vi "HFRR ADV v044.vi"() -> ()   [LabVIEW 2025] (continued)
              n2263 = Fract/Exp String To Number(string=w2652) -> (number=w2648:dbl)  [unwired: 3 in, 1 out]
              n2264 = Fract/Exp String To Number(string=w2642) -> (number=w2645:dbl)  [unwired: 3 in, 1 out]
              n2265 = Add(x=w2645, y=0.0) -> (x+y=w2641:dbl)
            }
            n2266 = Delete From Array(array=w2507, index=0) -> (array with subset deleted=w2480:dbl[])  [unwired: 1 in, 1 out]
            n2267 = Delete From Array(array=w2570, index=0) -> (array with subset deleted=w2543:dbl[])  [unwired: 1 in, 1 out]
            n2268 = Delete From Array(array=w2550, index=0) -> (array with subset deleted=w2538:dbl[])  [unwired: 1 in, 1 out]
            n2269 = Delete From Array(array=w2568, index=0) -> (array with subset deleted=w2569:dbl[])  [unwired: 1 in, 1 out]
            n2270 = call-poly <vilib>:"Mean.vi"("X"=w2480) -> ("mean"=→"КОФ2 4":dbl)  [unwired: 1 out]
            n2271 = call-poly <vilib>:"Mean.vi"("X"=w2543) -> ("mean"=→"КОФ3":dbl)  [unwired: 1 out]
            n2272 = call-poly <vilib>:"Mean.vi"("X"=w2538) -> ("mean"=→"CP3":dbl)  [unwired: 1 out]
            n2273 = Delete From Array(array=w2532, index=0) -> (array with subset deleted=w2459:dbl[])  [unwired: 1 in, 1 out]
            n2274 = Delete From Array(array=w2471, index=0) -> (array with subset deleted=w2458:dbl[])  [unwired: 1 in, 1 out]
            n2275 = Delete From Array(array=w2511, index=0) -> (array with subset deleted=w2482:dbl[])  [unwired: 1 in, 1 out]
            n2276 = Delete From Array(array=w2589, index=0) -> (array with subset deleted=w2544:dbl[])  [unwired: 1 in, 1 out]
            n2277 = Delete From Array(array=w2555, index=0) -> (array with subset deleted=w2540:dbl[])  [unwired: 1 in, 1 out]
            "array w/ subset deleted" <- w2540
            n2278 = Delete From Array(array=w2586, index=0) -> (array with subset deleted=w2587:dbl[])  [unwired: 1 in, 1 out]
            n2279 = call-poly <vilib>:"Mean.vi"("X"=w2482) -> ("mean"=→"КОФ2 2":dbl)  [unwired: 1 out]
            n2280 = call-poly <vilib>:"Mean.vi"("X"=w2544) -> ("mean"=→"КОФ1":dbl)  [unwired: 1 out]
            n2281 = Bundle "Bundle"(w2459, w2458) -> (w2464:cluster{dbl[], dbl[]})  [unwired: 1 in]
            n2282 = Bundle "Bundle"(w2459, w2587) -> (w2451:cluster{dbl[], dbl[]})  [unwired: 1 in]
            n2283 = Delete From Array(array=w2466, index=0) -> (array with subset deleted=w2454:dbl[])  [unwired: 1 in, 1 out]
            n2284 = Delete From Array(array=w2467, index=0) -> (array with subset deleted=w2456:dbl[])  [unwired: 1 in, 1 out]
            n2285 = Delete From Array(array=w2577, index=0) -> (array with subset deleted=w2578:dbl[])  [unwired: 1 in, 1 out]
            n2286 = Delete From Array(array=w2465, index=0) -> (array with subset deleted=w2452:dbl[])  [unwired: 1 in, 1 out]
            n2287 = Delete From Array(array=w2559, index=0) -> (array with subset deleted=w2560:dbl[])  [unwired: 1 in, 1 out]
            n2288 = Delete From Array(array=w2584, index=0) -> (array with subset deleted=w2490:dbl[])  [unwired: 1 in, 1 out]
            n2289 = Delete From Array(array=w2530, index=0) -> (array with subset deleted=w2486:dbl[])  [unwired: 1 in, 1 out]
            n2290 = Delete From Array(array=w2566, index=0) -> (array with subset deleted=w2488:dbl[])  [unwired: 1 in, 1 out]
            n2291 = Delete From Array(array=w2526, index=0) -> (array with subset deleted=w2484:dbl[])  [unwired: 1 in, 1 out]
            n2292 = Delete From Array(array=w2575, index=0) -> (array with subset deleted=w2489:dbl[])  [unwired: 1 in, 1 out]
            n2293 = Delete From Array(array=w2528, index=0) -> (array with subset deleted=w2485:dbl[])  [unwired: 1 in, 1 out]
            n2294 = Delete From Array(array=w2509, index=0) -> (array with subset deleted=w2481:dbl[])  [unwired: 1 in, 1 out]
            n2295 = Delete From Array(array=w2553, index=0) -> (array with subset deleted=w2539:dbl[])  [unwired: 1 in, 1 out]
            n2296 = Delete From Array(array=w2580, index=0) -> (array with subset deleted=w2541:dbl[])  [unwired: 1 in, 1 out]
            n2297 = Delete From Array(array=w2557, index=0) -> (array with subset deleted=w2487:dbl[])  [unwired: 1 in, 1 out]
            n2298 = Delete From Array(array=w2524, index=0) -> (array with subset deleted=w2483:dbl[])  [unwired: 1 in, 1 out]
            n2299 = Delete From Array(array=w2505, index=0) -> (array with subset deleted=w2479:dbl[])  [unwired: 1 in, 1 out]
            n2300 = Delete From Array(array=w2549, index=0) -> (array with subset deleted=w2537:dbl[])  [unwired: 1 in, 1 out]
            n2301 = Delete From Array(array=w2562, index=0) -> (array with subset deleted=w2542:dbl[])  [unwired: 1 in, 1 out]
            n2302 = Delete From Array(array=w2572, index=0) -> (array with subset deleted=w2455:dbl[])  [unwired: 1 in, 1 out]
            n2303 = Delete From Array(array=w2582, index=0) -> (array with subset deleted=w2457:dbl[])  [unwired: 1 in, 1 out]
            n2304 = Delete From Array(array=w2564, index=0) -> (array with subset deleted=w2453:dbl[])  [unwired: 1 in, 1 out]
            n2305 = Bundle "Bundle"(w2459, w2490) -> (w2477:cluster{dbl[], dbl[]})  [unwired: 1 in]
            n2306 = Bundle "Bundle"(w2459, w2544) -> (w2478:cluster{dbl[], dbl[]})  [unwired: 1 in]
            n2307 = Bundle "Bundle"(w2490, w2486) -> (w2492:cluster{dbl[], dbl[]})  [unwired: 1 in]
            n2308 = Bundle "Bundle"(w2455, w2454) -> (w2462:cluster{dbl[], dbl[]})  [unwired: 1 in]
            n2309 = Bundle "Bundle"(w2488, w2484) -> (w2494:cluster{dbl[], dbl[]})  [unwired: 1 in]
            n2310 = Bundle "Bundle"(w2455, w2488) -> (w2598:cluster{dbl[], dbl[]})  [unwired: 1 in]
            n2311 = Bundle "Bundle"(w2455, w2484) -> (w2522:cluster{dbl[], dbl[]})  [unwired: 1 in]
            n2312 = Bundle "Bundle"(w2455, w2543) -> (w2608:cluster{dbl[], dbl[]})  [unwired: 1 in]
            n2313 = Bundle "Bundle"(w2455, w2538) -> (w2546:cluster{dbl[], dbl[]})  [unwired: 1 in]
            n2314 = Bundle "Bundle"(w2455, w2569) -> (w2593:cluster{dbl[], dbl[]})  [unwired: 1 in]
            n2315 = Bundle "Bundle"(w2489, w2485) -> (w2493:cluster{dbl[], dbl[]})  [unwired: 1 in]
            n2316 = Bundle "Bundle"(w2457, w2456) -> (w2463:cluster{dbl[], dbl[]})  [unwired: 1 in]
            n2317 = Bundle "Bundle"(w2457, w2489) -> (w2600:cluster{dbl[], dbl[]})  [unwired: 1 in]
            n2318 = Bundle "Bundle"(w2457, w2485) -> (w2523:cluster{dbl[], dbl[]})  [unwired: 1 in]
            n2319 = Bundle "Bundle"(w2457, w2539) -> (w2547:cluster{dbl[], dbl[]})  [unwired: 1 in]
            n2320 = Bundle "Bundle"(w2457, w2541) -> (w2609:cluster{dbl[], dbl[]})  [unwired: 1 in]
            n2321 = Bundle "Bundle"(w2457, w2578) -> (w2591:cluster{dbl[], dbl[]})  [unwired: 1 in]
            n2322 = Bundle "Bundle"(w2487, w2483) -> (w2495:cluster{dbl[], dbl[]})  [unwired: 1 in]
            n2323 = Bundle "Bundle"(w2453, w2452) -> (w2461:cluster{dbl[], dbl[]})  [unwired: 1 in]
            n2324 = Bundle "Bundle"(w2453, w2487) -> (w2599:cluster{dbl[], dbl[]})  [unwired: 1 in]
            n2325 = Bundle "Bundle"(w2453, w2483) -> (w2521:cluster{dbl[], dbl[]})  [unwired: 1 in]
            n2326 = Bundle "Bundle"(w2453, w2537) -> (w2545:cluster{dbl[], dbl[]})  [unwired: 1 in]
            n2327 = Bundle "Bundle"(w2453, w2542) -> (w2607:cluster{dbl[], dbl[]})  [unwired: 1 in]
            n2328 = Bundle "Bundle"(w2453, w2560) -> (w2592:cluster{dbl[], dbl[]})  [unwired: 1 in]
            n2329 = call-poly <vilib>:"Mean.vi"("X"=w2540) -> ("mean"=→"CP1":dbl)  [unwired: 1 out]
            n2330 = call-poly <vilib>:"Mean.vi"("X"=w2481) -> ("mean"=→"КОФ2 3":dbl)  [unwired: 1 out]
            n2331 = call-poly <vilib>:"Mean.vi"("X"=w2539) -> ("mean"=→"CP2":dbl)  [unwired: 1 out]
            n2332 = call-poly <vilib>:"Mean.vi"("X"=w2541) -> ("mean"=→"КОФ2":dbl)  [unwired: 1 out]
            n2333 = call-poly <vilib>:"Mean.vi"("X"=w2479) -> ("mean"=→"КОФ2 5":dbl)  [unwired: 1 out]
            n2334 = call-poly <vilib>:"Mean.vi"("X"=w2537) -> ("mean"=→"CP4":dbl)  [unwired: 1 out]
            n2335 = call-poly <vilib>:"Mean.vi"("X"=w2542) -> ("mean"=→"КОФ4":dbl)  [unwired: 1 out]
            n2336 = Bundle "Bundle"(w2459, w2486) -> (w2450:cluster{dbl[], dbl[]})  [unwired: 1 in]
            n2337 = Bundle "Bundle"(w2459, w2540) -> (w2473:cluster{dbl[], dbl[]})  [unwired: 1 in]
            n2338 = Build Array "Build Array"(w2450, w2473) -> (w2476:cluster{dbl[], dbl[]}[])
            "XY Graph 17" <- w2476
            n2339 = Build Array "Build Array"(w2464, w2463, w2462, w2461) -> (→"Frequency ( Hz )":cluster{dbl[], dbl[]}[])
            n2340 = Build Array "Build Array"(w2492, w2493, w2494, w2495) -> (→"Air Temp ( °C ) vs Humidity ( % RH )":cluster{dbl[], dbl[]}[])
            n2341 = Build Array "Build Array"(w2477, w2600, w2598, w2599) -> (→"Air Temperature  ( °C )":cluster{dbl[], dbl[]}[])
            n2342 = Build Array "Build Array"(w2450, w2523, w2522, w2521) -> (→"Humidity ( %RH )":cluster{dbl[], dbl[]}[])
            n2343 = Build Array "Build Array"(w2478, w2609, w2608, w2607) -> (→"Coefficient Of Friction":cluster{dbl[], dbl[]}[])
            n2344 = Build Array "Build Array"(w2473, w2547, w2546, w2545) -> (→"Sample Temperature ( °C )":cluster{dbl[], dbl[]}[])
            n2345 = Build Array "Build Array"(w2451, w2591, w2593, w2592) -> (→"XY Graph 13":cluster{dbl[], dbl[]}[])
            n2346 = Bundle "Bundle"(w2459, w2482) -> (w2504:cluster{dbl[], dbl[]})  [unwired: 1 in]
            n2347 = Bundle "Bundle"(w2455, w2480) -> (w2502:cluster{dbl[], dbl[]})  [unwired: 1 in]
            n2348 = Bundle "Bundle"(w2457, w2481) -> (w2503:cluster{dbl[], dbl[]})  [unwired: 1 in]
            n2349 = Bundle "Bundle"(w2453, w2479) -> (w2501:cluster{dbl[], dbl[]})  [unwired: 1 in]
            n2350 = Build Array "Build Array"(w2504, w2503, w2502, w2501) -> (→"Stroke ( mm )":cluster{dbl[], dbl[]}[])
            n2351 = local write "XY Graph 16"(w2476) -> ()
          }
          frame #2 {
          }
          frame #3 {
            n2352 = local write "Numeric 8"(0 ("Numeric 8")) -> ()
            n2353 = local write "Numeric 11"(0 ("Numeric 11")) -> ()
            n2354 = local write "Numeric 12"(0 ("Numeric 12")) -> ()
            n2355 = local write "Numeric 13"(0 ("Numeric 13")) -> ()
            n2356 = property on="OPEN" class="Bool (strict)"("Visible"=TRUE) -> ()  [unwired: 2 in, 2 out]
            n2357 = local read "String Control 2"() -> (w2776:string)
            n2358 = local read "String Control 4"() -> (w2775:string)
            n2359 = local read "String Control 6"() -> (w2774:string)
            n2360 = local read "String Control 8"() -> (w2773:string)
            n2361 = Match Pattern(string=w2776, regular expression="Samples / cycle :- ") -> (after substring=w2790:string)  [unwired: 1 in, 3 out]
            n2362 = Match Pattern(string=w2776, regular expression="Frequency :- ") -> (after substring=w2809:string)  [unwired: 1 in, 3 out]
            n2363 = Match Pattern(string=w2775, regular expression="Samples / cycle :- ") -> (after substring=w2786:string)  [unwired: 1 in, 3 out]
            n2364 = Match Pattern(string=w2775, regular expression="Frequency :- ") -> (after substring=w2804:string)  [unwired: 1 in, 3 out]
            n2365 = Match Pattern(string=w2774, regular expression="Samples / cycle :- ") -> (after substring=w2782:string)  [unwired: 1 in, 3 out]
            n2366 = Match Pattern(string=w2774, regular expression="Frequency :- ") -> (after substring=w2799:string)  [unwired: 1 in, 3 out]
            n2367 = Match Pattern(string=w2773, regular expression="Samples / cycle :- ") -> (after substring=w2778:string)  [unwired: 1 in, 3 out]
            n2368 = Match Pattern(string=w2773, regular expression="Frequency :- ") -> (after substring=w2794:string)  [unwired: 1 in, 3 out]
            n2369 = String Subset(string=w2790, length (rest)=6 ("length (rest)")) -> (substring=w2792:string)  [unwired: 1 in]
            n2370 = String Subset(string=w2809, length (rest)=9 ("length (rest)")) -> (substring=w2811:string)  [unwired: 1 in]
            n2371 = String Subset(string=w2786, length (rest)=6 ("length (rest)")) -> (substring=w2788:string)  [unwired: 1 in]
            n2372 = String Subset(string=w2804, length (rest)=9 ("length (rest)")) -> (substring=w2806:string)  [unwired: 1 in]
            n2373 = String Subset(string=w2782, length (rest)=6 ("length (rest)")) -> (substring=w2784:string)  [unwired: 1 in]
            n2374 = String Subset(string=w2799, length (rest)=9 ("length (rest)")) -> (substring=w2801:string)  [unwired: 1 in]
            n2375 = String Subset(string=w2778, length (rest)=6 ("length (rest)")) -> (substring=w2780:string)  [unwired: 1 in]
            n2376 = String Subset(string=w2794, length (rest)=9 ("length (rest)")) -> (substring=w2796:string)  [unwired: 1 in]
            n2377 = Fract/Exp String To Number(string=w2792) -> (number=w2772:dbl)  [unwired: 3 in, 1 out]
            n2378 = Fract/Exp String To Number(string=w2811) -> (number=w2812:dbl)  [unwired: 3 in, 1 out]
            n2379 = Fract/Exp String To Number(string=w2788) -> (number=w2771:dbl)  [unwired: 3 in, 1 out]
            n2380 = Fract/Exp String To Number(string=w2806) -> (number=w2807:dbl)  [unwired: 3 in, 1 out]
            n2381 = Fract/Exp String To Number(string=w2784) -> (number=w2770:dbl)  [unwired: 3 in, 1 out]
            n2382 = Fract/Exp String To Number(string=w2801) -> (number=w2802:dbl)  [unwired: 3 in, 1 out]
            n2383 = Fract/Exp String To Number(string=w2780) -> (number=w2769:dbl)  [unwired: 3 in, 1 out]
            n2384 = Fract/Exp String To Number(string=w2796) -> (number=w2797:dbl)  [unwired: 3 in, 1 out]
            n2385 = local write "sample1"(w2772) -> ()
            n2386 = local write "freq1"(w2812) -> ()
            n2387 = local write "sample2"(w2771) -> ()
            n2388 = local write "freq2"(w2807) -> ()
            n2389 = local write "sample3"(w2770) -> ()
            n2390 = local write "freq3"(w2802) -> ()
            n2391 = local write "sample4"(w2769) -> ()
            n2392 = local write "freq 4"(w2797) -> ()
          }
        }
      }
    }
    n2393 = case shown="True" w2370 {
      selector: w2370 -> [_ w2389]
      frame False {
      }
      frame True {
        n2394 = Not(x=w2389) -> (.not. x?=w2385:bool)
        n2395 = local write "service 3"(w2385) -> ()
        n2396 = local write "OPEN 6"(w2385) -> ()
        n2397 = call <vilib>:"System Exec.vi"("wait until completion? (T)"=TRUE, "command line"="C:\\LAB-IQ\\Scar View.exe") -> ("error out"=→"error out 5":errorcluster)  [unwired: 6 in, 3 out]
      }
    }
    n2398 = case shown="\"Acquire\", Default" w2379 {
      frame "Acquire", Default {
        # "Elapsed time\ncof\nstroke\nAir temp\nTemp\nHumidity"
        n2399 = disable-structure shown="Disabled" {
          frame Disabled {
            n2400 = local read "Flag"() -> (w3088:dbl)
            n2401 = local read "RUN"() -> (w3085:bool)
            n2402 = Not(x=w3085) -> (.not. x?=w3084:bool)
            n2403 = Equal?(x=w3088, y=10.0) -> (x = y?=w3086:bool)
            n2404 = And(x=w3086, y=w3084) -> (x .and. y?=w3083:bool)
            n2405 = case shown="True" w3083 {
              frame False {
              }
              frame True {
                w3089 = FALSE ("Heater Button")
                n2406 = local write "Humidity"(w3089) -> ()
                n2407 = local write "Heater Button"(w3089) -> ()
              }
            }
          }
          frame Enabled {
          }
        }
        n2408 = disable-structure shown="Disabled" {
          frame Disabled {
            n2409 = case shown="True" {
              selector: _ -> [_ _]
              frame False {
              }
              frame True {
                w3134 = TRUE ("Heater")
                n2410 = local write "Humidity"(w3134) -> ()
                n2411 = local write "Heater Button"(w3134) -> ()
                n2412 = local read "TEST STANDARD"() -> (w3137:T5)
                n2413 = local read "TEST STANDARD"() -> (w3132:T5)
                n2414 = Equal?(x=w3137, y=enum16{"ASTM D6079", "ISO 12156", "Custom"}."ISO 12156" ("Test Standard")) -> (x = y?=w3135:bool)
                n2415 = Equal?(x=w3132, y=enum16{"ASTM D6079", "ISO 12156", "Custom"}."ASTM D6079" ("Test Standard")) -> (x = y?=w3131:bool)
                n2416 = case shown="True" w3135 {
                  frame False {
                  }
                  frame True {
                    n2417 = local write "airtempflg"(FALSE ("airtempflg")) -> ()
                    n2418 = local write item#-1(TRUE ("Heater")) -> ()
                  }
                }
                n2419 = case shown="True" w3131 {
                  frame False {
                  }
                  frame True {
                    n2420 = local write "airtempflg"(TRUE ("airtempflg")) -> ()
                    n2421 = local write item#-1(FALSE ("Heater")) -> ()
                  }
                }
              }
            }
          }
          frame Enabled {
          }
        }
        n2422 = stacked-sequence {
          frame #0 {
            n2423 = case shown="True" "RST FF" {
              frame False {
              }
              frame True {
                w3151 = 0.0 ("X Scale.Range:Maximum")
                n2424 = property on="Frictional Force ( N )" class="WFChart (strict)"("XScale.Maximum"=600.0 ("X Scale.Range:Maximum"), "XScale.Minimum"=w3151, "YScale.Maximum"=10.0 ("Y Scale.Range:Maximum"), "YScale.Minimum"=w3151) -> ()  [unwired: 2 in, 2 out]
              }
            }
          }
          frame #1 {
            n2425 = case shown="True" "RST TEMP" {
              frame False {
              }
              frame True {
                n2426 = property on="Temperature ( Deg C )" class="WFChart (strict)"("XScale.Minimum"=0.0 ("X Scale.Range:Minimum"), "XScale.Maximum"=600.0 ("X Scale.Range:Maximum"), "YScale.Minimum"=0.0 ("Y Scale.Range:Minimum"), "YScale.Maximum"=100.0 ("Y Scale.Range:Maximum")) -> ()  [unwired: 2 in, 2 out]
              }
            }
          }
          frame #2 {
            n2427 = case shown="True" "RSTCOF" {
              frame False {
              }
              frame True {
                n2428 = property on="Coefficient of Friction" class="WFChart (strict)"("XScale.Minimum"=0.0 ("X Scale.Range:Minimum"), "XScale.Maximum"=600.0 ("X Scale.Range:Maximum"), "YScale.Maximum"=1.0 ("X Scale.Range:Minimum"), "YScale.Minimum"=0.0 ("X Scale.Range:Minimum")) -> ()  [unwired: 2 in, 2 out]
              }
            }
          }
          frame #3 {
            n2429 = case shown="True" "RSTCOF 2" {
              frame False {
              }
              frame True {
                (unwired) 100.0 ("Y Scale.Range:Maximum")
                (unwired) 0.0 ("Y Scale.Range:Minimum")
                (unwired) 600.0 ("X Scale.Range:Maximum")
                (unwired) 0.0 ("X Scale.Range:Minimum")
              }
            }
          }
          frame #4 {
            n2430 = case shown="True" "RSTCOF 3" {
              frame False {
              }
              frame True {
                n2431 = property on="Electrical Contact Resistance ( % )" class="WFChart (strict)"("XScale.Minimum"=0.0 ("X Scale.Range:Minimum"), "XScale.Maximum"=600.0 ("X Scale.Range:Maximum"), "YScale.Minimum"=0.0 ("Y Scale.Range:Minimum"), "YScale.Maximum"=100.0 ("Y Scale.Range:Maximum")) -> ()  [unwired: 2 in, 2 out]
              }
            }
          }
        }
        n2432 = local read "RUN"() -> (w3078:bool)
        n2433 = case shown="False" w3078 {
          frame False {
          }
          frame True {
          }
        }
        n2434 = local read "RUN"() -> (w3082:bool)
        n2435 = case shown="False" w3082 {
          tunnel: [FALSE ("TEST RUNNING") TRUE ("TEST RUNNING")] -> w3081
          frame False {
            w3170 = 0.0 ("Flag")
            n2436 = local write "Elapsed time"(0.0 ("elapsedtime")) -> ()
            n2437 = local write "Time Remaining"(w3170) -> ()
            n2438 = local write "Flag"(w3170) -> ()
            n2439 = local write "Remaining Time"(w3170) -> ()
          }
          frame True {
            n2440 = local write "Flag"(10.0 ("Flag")) -> ()
          }
        }
        n2441 = local read "AIR TEMP"() -> (w3076:dbl)
        n2442 = Greater Or Equal?(x=w3076, y=15.0) -> (x >= y?=w3077:bool)
        "powstat" <- w3077
        n2443 = case shown="True" "Save & Continue" {
          frame False {
          }
          frame True {
            n2444 = local read "USER ID"() -> (w3474:string)
            n2445 = local read "FILE"() -> (w3482:string)
            n2446 = String Length(string=w3482) -> (length=w3480:i32)
            n2447 = String Length(string=w3474) -> (length=w3477:i32)
            n2448 = Greater?(x=w3480, y=0) -> (0:w3479:bool)
            n2449 = Greater?(x=w3477, y=0) -> (0:w3476:bool)
            n2450 = And(x=w3479, y=w3476) -> (x .and. y?=w3475:bool)
            n2451 = case shown="True" w3475 {
              frame False {
                n2452 = stacked-sequence {
                  frame #0 {
                    n2453 = One Button Dialog(message="Please Enter a File Name and Operator ID to save data !", button name ("OK")="Ok") -> ()  [unwired: 1 out]
                  }
                  frame #1 {
                    n2454 = local write "Save & Continue"(FALSE ("OK Button")) -> ()
                  }
                }
                n2455 = local write "Save & Continue"(FALSE ("OK Button")) -> ()
              }
              frame True {
                n2456 = stacked-sequence {
                  frame #0 {
                    n2457 = local read "FILE"() -> (w3488:string)
                    n2458 = call "file check.vi"("file name in"=w3488) -> ("file name out"=w3487:string)  [unwired: 9 in, 1 out]
                    n2459 = call <vilib>:"Application Directory.vi"() -> ("Application Directory"=w3498:path)
                    n2460 = Build Path(base path=w3498, name or relative path="data") -> (appended path=w3497:path)
                    n2461 = call <vilib>:"Trim Whitespace.vi"("string"=w3487) -> ("trimmed string"=w3495:string)  [unwired: 1 in]
                    n2462 = call <vilib>:"Trim Whitespace.vi"("string"=w3487) -> ("trimmed string"=w3496:string)  [unwired: 1 in]
                    n2463 = List Folder(path=w3497) -> (folder names=w3493:string[])  [unwired: 3 in, 3 out]
                    n2464 = Match Pattern(string=w3495, regular expression="_(") -> (before substring=w3492:string)  [unwired: 1 in, 3 out]
                    n2465 = for {
                      tunnel: w3493 -> [w3507] mode=indexing
                      tunnel: w3492 -> [w3505]
                      shift-right: [w3503] -> w3490
                      shift-left: bool[] [] -> [w3504]
                      n2466 = Match Pattern(string=w3507, regular expression="_(") -> (before substring=w3506:string)  [unwired: 1 in, 3 out]
                      n2467 = Equal?(x=w3506, y=w3505) -> (x = y?=w3502:bool)
                      n2468 = case shown="True" w3502 {
                        tunnel: w3502 -> [_ w3510]
                        tunnel: w3504 -> [w3509 w3512]
                        tunnel: [w3509 w3511] -> w3503
                        frame False {
                        }
                        frame True {
                          n2469 = Insert Into Array(array=w3512, new element=w3510) -> (w3511:bool[])  [unwired: 1 in]
                        }
                      }
                    }
                    n2470 = Equal?(x=w3493, y=w3492) -> (x = y?=w3501:bool[])
                    n2471 = Or Array Elements(Boolean array=w3501) -> (logical OR=w3500:bool)
                    n2472 = Array Size(array=w3490) -> (size(s)=w3489:i32)
                    n2473 = case shown="True" w3500 {
                      tunnel: w3496 -> [_ w3520]
                      tunnel: w3489 -> [_ w3513]
                      frame False {
                      }
                      frame True {
                        n2474 = Number To Decimal String(number=w3513) -> (decimal integer string=w3516:string)  [unwired: 1 in]
                        n2475 = Search/Split String(string=w3520, search string/char (-)="_(" ("regular expression")) -> (substring before match=w3518:string)  [unwired: 1 in, 2 out]
                        n2476 = Concatenate Strings(w3518, "_(" ("regular expression"), w3516, ")" ("regular expression")) -> (w3514:string)
                        n2477 = local write "FILE"(w3514) -> ()
                      }
                    }
                  }
                  frame #1 {
                    w3523 = 0.0
                    w3536 = cluster{"y":dbl, dbl, "y":dbl}[] [] ("History Data")
                    w3537 = FALSE ("Heater Button")
                    (unwired) ")!" ("string")
                    (unwired) ")" ("string")
                    w3535 = dbl[] [] ("History Data")
                    w3541 = "\r"
                    # "C:\\WinDucom\\Data\\"
                    # "C:\\LAB-IQ-NXT\\data"
                    n2478 = local write "Humidity ( %RH )"(w3523) -> ()
                    n2479 = local write "Frequency ( Hz )"(w3523) -> ()
                    n2480 = local write "Stroke 3"(w3523) -> ()
                    n2481 = local write "speedop"(0.0 ("PIDclk 2")) -> ()
                    n2482 = local write "Set Temp 2"(65.0 ("Set Temp 2")) -> ()
                    n2483 = local write "AIR TEMP"(w3523) -> ()
                    n2484 = local write "clk"(0.0 ("clk")) -> ()
                    n2485 = local write "Stroke 4"(w3523) -> ()
                    n2486 = local write "COF 2"(w3523) -> ()
                    n2487 = local write "TEMP"(w3523) -> ()
                    n2488 = local write "ecr 3"(w3523) -> ()
                    n2489 = local write "FF 3"(w3523) -> ()
                    n2490 = local write "FF 2"(w3523) -> ()
                    n2491 = property on="Coefficient of Friction" class="WFChart (strict)"("History Data"=w3535) -> ()  [unwired: 2 in, 2 out]
                    n2492 = property on="Coefficient of Friction" class="WFChart (strict)"("History Data"=w3535) -> ()  [unwired: 2 in, 2 out]
                    n2493 = property on="Frictional Force ( N )" class="WFChart (strict)"("History Data"=w3535) -> ()  [unwired: 2 in, 2 out]
                    n2494 = property on="Electrical Contact Resistance ( % )" class="WFChart (strict)"("History Data"=w3535) -> ()  [unwired: 2 in, 2 out]
                    n2495 = property on="Electrical Contact Resistance ( % )" class="WFChart (strict)"("History Data"=w3535) -> ()  [unwired: 2 in, 2 out]
                    n2496 = property on="Temperature ( Deg C )" class="WFChart (strict)"("History Data"=w3535) -> ()  [unwired: 2 in, 2 out]
                    n2497 = property on="Frictional Force ( N )" class="WFChart (strict)"("History Data"=w3535) -> ()  [unwired: 2 in, 2 out]
                    n2498 = property on="Coefficient of Friction" class="WFChart (strict)"("History Data"=w3535) -> ()  [unwired: 2 in, 2 out]
                    n2499 = property on="Frictional Force ( N )" class="WFChart (strict)"("History Data"=w3535) -> ()  [unwired: 2 in, 2 out]
                    n2500 = property on="Electrical Contact Resistance ( % )" class="WFChart (strict)"("History Data"=w3535) -> ()  [unwired: 2 in, 2 out]
                    n2501 = property on="Temperature ( Deg C )" class="WFChart (strict)"("History Data"=w3535) -> ()  [unwired: 2 in, 2 out]
                    n2502 = property on="Stroke ( mm )" class="WFChart (strict)"("History Data"=w3536) -> ()  [unwired: 2 in, 2 out]
                    n2503 = property on="Stroke ( mm )" class="WFChart (strict)"("History Data"=w3536) -> ()  [unwired: 2 in, 2 out]
                    n2504 = local write "Humidity"(w3537) -> ()
                    n2505 = local write "Heater Button"(w3537) -> ()
                    n2506 = local read "FILE"() -> (w3531:string)
                    n2507 = disable-structure shown="Enabled" {
                      disable-tunnel: [w3575 _] -> w3522
                      frame Enabled {
                        n2508 = local read "NORMAL LOAD"() -> (w3575:dbl)
                      }
                      frame Disabled {
                      }
                    }
                    n2509 = call "file check.vi"("file name in"=w3531) -> ("error out"=w3534:errorcluster, "file name out"=w3528:string)  [unwired: 9 in]
                    n2510 = call "FILE PATH CREATION.vi"("error in"=w3534, "FILE NAME :"=w3528) -> ("FILE OUT"=w3527:path)  [unwired: 8 in, 1 out]
                    n2511 = Concatenate Strings(w3528, ".dgf" ("Substring")) -> (w3533:string)
                    n2512 = Concatenate Strings(w3528, ".duf" ("Substring")) -> (w3529:string)
                    n2513 = Multiply(x=w3522, y=1.0) -> (x*y=w3554:dbl)
                    n2514 = Build Path(base path=w3527, name or relative path=w3533) -> (appended path=w3526:path)
                    n2515 = Build Path(base path=w3527, name or relative path=w3529) -> (appended path=w3525:path)
                    n2516 = Number To Fractional String(number=w3554, width (-)=i16 5, precision (6)=i16 2) -> (F-format string=w3562:string)  [unwired: 1 in]
                    n2517 = local read "tested by"() -> (w3521:string)
                    n2518 = local read "Fuel Discription :"() -> (w3550:string)
                    n2519 = local read "Batch Ref Num :"() -> (w3539:string)
                    n2520 = Get Date/Time String(date format (0)=enum16{"short", "long", "abbreviated"}."short") -> (date string=w3573:string, time string=w3570:string)  [unwired: 2 in]
                    n2521 = local read "Remarks :"() -> (w3549:string)
                    n2522 = Concatenate Strings("Load :- " ("Substring"), w3562, " grams ," ("Substring")) -> (w3561:string)
                    n2523 = local read "String 41"() -> (w3542:string)
                    n2524 = Concatenate Strings(w3550) -> (w3551:string)
                    n2525 = Concatenate Strings(w3539) -> (w3538:string)
                    n2526 = Concatenate Strings(w3521) -> (w3545:string)
                    n2527 = Concatenate Strings("(" ("Substring"), w3573, ")" ("Substring"), w3570) -> (w3544:string)
                    "concatenated string" <- w3544
                    n2528 = Concatenate Strings(w3549, "," ("string")) -> (w3548:string)
                    n2529 = Concatenate Strings("  TIME;      COF;       STROKE;     AIR TEMP;  TEMP;  HUMIDITY;  ECR; PID-OUT; FREQUENCY" ("Substring"), "\r") -> (w3557:string)
                    n2530 = Concatenate Strings(w3542, w3541, "Fuel Discription :-" ("Substring"), w3551, w3541, w3561, w3541, "Batch Ref Num :-" ("Substring"), w3538, w3541, " Remarks :- " ("Substring"), w3548, w3541, " Date :- " ("Substring"), w3544, w3541, "Tested By :-" ("Substring"), w3545) -> (w3555:string)
                    "REMARKS" <- w3555
                    n2531 = call <vilib>:"Write Characters To File.vi"("append to file? (new file:F)"=FALSE, "character string"=w3557, "file path (dialog if empty)"=w3526) -> ()  [unwired: 2 in, 1 out]
                    n2532 = call <vilib>:"Write Characters To File.vi"("append to file? (new file:F)"=FALSE, "character string"=w3555, "file path (dialog if empty)"=w3525) -> ()  [unwired: 2 in, 1 out]
                  }
                  frame #2 {
                    n2533 = local write "Cycles elapsed"(0 ("Cycles elapsed")) -> ()
                    n2534 = local write "cyclecount"(0 ("cyclecount")) -> ()
                    n2535 = local write "Save & Continue"(FALSE ("OK")) -> ()
                    n2536 = local write "autostrtflg"(TRUE ("autostrtflg")) -> ()
                    n2537 = local write "Save"(FALSE ("Save")) -> ()
                    n2538 = Get Date/Time In Seconds() -> (seconds since 1Jan1904=w3580:timestamp)
                    n2539 = To Double Precision Float(number=w3580) -> (double precision float=w3579:dbl)
                    n2540 = local write "acq timer"(w3579) -> ()
                    n2541 = One Button Dialog(message="Please ensure sample is mounted properly and machine is ready in all aspects for testing !", button name ("OK")="Ok") -> ()  [unwired: 1 out]
                  }
                  frame #3 {
                    n2542 = stacked-sequence {
                      frame #0 {
                        n2543 = local write "Main Dashboard Buttons"(T1."Dashboard" ("Main Dashboard Buttons")) -> ()
                        n2544 = local write "Main Tab"(T4."Acquire" ("Main Tab")) -> ()
                      }
                      frame #1 {
                        n2545 = local write "EVENT LOG"("" ("EVENT LOG")) -> ()
                      }
                      frame #2 {
                        n2546 = Wait (ms)(milliseconds to wait=u32 50) -> ()  [unwired: 1 out]
                      }
                      frame #3 {
                        n2547 = disable-structure shown="Disabled" {
                          frame Disabled {
                            n2548 = local read "EVENT LOG"() -> (w3592:string)
                            n2549 = call "Event Log.vi"("Content"="Test Details", "EVENT LOG"=w3592) -> ("EVENT LOG"=w3591:string)  [unwired: 8 in, 1 out]
                            n2550 = local write "EVENT LOG"(w3591) -> ()
                          }
                          frame Enabled {
                          }
                        }
                      }
                      frame #4 {
                        n2551 = Wait (ms)(milliseconds to wait=u32 50) -> ()  [unwired: 1 out]
                      }
                      frame #5 {
                        n2552 = local read "FILE"() -> (w3594:string)
                        n2553 = Concatenate Strings("File Name :" ("Content"), w3594) -> (w3595:string)
                        n2554 = local read "EVENT LOG"() -> (w3598:string)
                        n2555 = call "Event Log.vi"("Content"=w3595, "EVENT LOG"=w3598) -> ("EVENT LOG"=w3597:string)  [unwired: 8 in, 1 out]
                        n2556 = local write "EVENT LOG"(w3597) -> ()
                      }
                      frame #6 {
                        n2557 = Wait (ms)(milliseconds to wait=u32 50) -> ()  [unwired: 1 out]
                      }
                      frame #7 {
                        n2558 = local read "Batch Ref Num :"() -> (w3600:string)
                        n2559 = Concatenate Strings("Batch Ref No :" ("Content"), w3600) -> (w3601:string)
                        n2560 = local read "EVENT LOG"() -> (w3604:string)
                        n2561 = call "Event Log.vi"("Content"=w3601, "EVENT LOG"=w3604) -> ("EVENT LOG"=w3603:string)  [unwired: 8 in, 1 out]
                        n2562 = local write "EVENT LOG"(w3603) -> ()
                      }
                      frame #8 {
                        n2563 = Wait (ms)(milliseconds to wait=u32 50) -> ()  [unwired: 1 out]
                      }
                      frame #9 {
                        n2564 = local read "tested by"() -> (w3606:string)
                        n2565 = Concatenate Strings("Tested By :" ("Content"), w3606) -> (w3607:string)
                        n2566 = local read "EVENT LOG"() -> (w3610:string)
                        n2567 = call "Event Log.vi"("Content"=w3607, "EVENT LOG"=w3610) -> ("EVENT LOG"=w3609:string)  [unwired: 8 in, 1 out]
                        n2568 = local write "EVENT LOG"(w3609) -> ()
                      }
                      frame #10 {
                        n2569 = Wait (ms)(milliseconds to wait=u32 50) -> ()  [unwired: 1 out]
                      }
                      frame #11 {
                        n2570 = local read "TEST STANDARD"() -> (w3613:T5)
                        n2571 = case shown="\"ASTM D6079\", Default" w3613 {
                          tunnel: ["ASTM D6079" "ISO 12156" "CEC F-096-A-06" "Custom"] -> w3612
                          frame "ASTM D6079", Default {
                          }
                          frame "ISO 12156" {
                          }
                          frame "CEC F-096-A-06" {
                          }
                          frame "Custom" {
                          }
                        }
                        n2572 = Concatenate Strings("Test Standard :" ("Content"), w3612) -> (w3614:string)
                        n2573 = local read "EVENT LOG"() -> (w3617:string)
                        n2574 = call "Event Log.vi"("Content"=w3614, "EVENT LOG"=w3617) -> ("EVENT LOG"=w3616:string)  [unwired: 8 in, 1 out]
                        n2575 = local write "EVENT LOG"(w3616) -> ()
                      }
                      frame #12 {
                        n2576 = Wait (ms)(milliseconds to wait=u32 50) -> ()  [unwired: 1 out]
                      }
                      frame #13 {
                        n2577 = local read "Fuel Discription :"() -> (w3623:string)
                        n2578 = Concatenate Strings("Fuel Description :" ("Content"), w3623) -> (w3624:string)
                        n2579 = local read "EVENT LOG"() -> (w3627:string)
                        n2580 = call "Event Log.vi"("Content"=w3624, "EVENT LOG"=w3627) -> ("EVENT LOG"=w3626:string)  [unwired: 8 in, 1 out]
                        n2581 = local write "EVENT LOG"(w3626) -> ()
                      }
                      frame #14 {
                        n2582 = Wait (ms)(milliseconds to wait=u32 50) -> ()  [unwired: 1 out]
                      }
                      frame #15 {
                        n2583 = local read "Remarks :"() -> (w3629:string)
                        n2584 = Concatenate Strings("Remarks :" ("Content"), w3629) -> (w3630:string)
                        n2585 = local read "EVENT LOG"() -> (w3633:string)
                        n2586 = call "Event Log.vi"("Content"=w3630, "EVENT LOG"=w3633) -> ("EVENT LOG"=w3632:string)  [unwired: 8 in, 1 out]
                        n2587 = local write "EVENT LOG"(w3632) -> ()
                      }
                      frame #16 {
                        n2588 = Wait (ms)(milliseconds to wait=u32 50) -> ()  [unwired: 1 out]
                      }
                      frame #17 {
                        n2589 = local read "USER ID"() -> (w3635:string)
                        n2590 = Concatenate Strings("Operator ID :" ("Content"), w3635) -> (w3637:string)
                        n2591 = local read "EVENT LOG"() -> (w3639:string)
                        n2592 = call "Event Log.vi"("Content"=w3637, "EVENT LOG"=w3639) -> ("EVENT LOG"=w3638:string)  [unwired: 8 in, 1 out]
                        n2593 = local write "EVENT LOG"(w3638) -> ()
                      }
                      frame #18 {
                        n2594 = Wait (ms)(milliseconds to wait=u32 50) -> ()  [unwired: 1 out]
                      }
                      frame #19 {
                        n2595 = disable-structure shown="Disabled" {
                          frame Disabled {
                            n2596 = local read "EVENT LOG"() -> (w3643:string)
                            n2597 = call "Event Log.vi"("Content"="Test Parameter", "EVENT LOG"=w3643) -> ("EVENT LOG"=w3642:string)  [unwired: 8 in, 1 out]
                            n2598 = local write "EVENT LOG"(w3642) -> ()
                          }
                          frame Enabled {
                          }
                        }
                      }
                      frame #20 {
                        n2599 = Wait (ms)(milliseconds to wait=u32 50) -> ()  [unwired: 1 out]
                      }
                      frame #21 {
                        n2600 = local read "Set Hz"() -> (w3647:dbl)
                        n2601 = Number To Fractional String(number=w3647, precision (6)=i16 2) -> (F-format string=w3646:string)  [unwired: 2 in]
                        n2602 = Concatenate Strings("Set Frequency [Hz] :" ("Content"), w3646) -> (w3649:string)
                        n2603 = local read "EVENT LOG"() -> (w3651:string)
                        n2604 = call "Event Log.vi"("Content"=w3649, "EVENT LOG"=w3651) -> ("EVENT LOG"=w3650:string)  [unwired: 8 in, 1 out]
                        n2605 = local write "EVENT LOG"(w3650) -> ()
                      }
                      frame #22 {
                        n2606 = Wait (ms)(milliseconds to wait=u32 50) -> ()  [unwired: 1 out]
                      }
                      frame #23 {
                        n2607 = local read "NORMAL LOAD"() -> (w3654:dbl)
                        n2608 = Number To Fractional String(number=w3654, precision (6)=i16 2) -> (F-format string=w3655:string)  [unwired: 2 in]
                        n2609 = Concatenate Strings("Applied Load [grams] :" ("Content"), w3655) -> (w3657:string)
                        n2610 = local read "EVENT LOG"() -> (w3659:string)
                        n2611 = call "Event Log.vi"("Content"=w3657, "EVENT LOG"=w3659) -> ("EVENT LOG"=w3658:string)  [unwired: 8 in, 1 out]
                        n2612 = local write "EVENT LOG"(w3658) -> ()
                      }
                      frame #24 {
                        n2613 = Wait (ms)(milliseconds to wait=u32 50) -> ()  [unwired: 1 out]
                      }
                      frame #25 {
                        n2614 = local read "Set Strk"() -> (w3662:dbl)
                        n2615 = Number To Fractional String(number=w3662, precision (6)=i16 2) -> (F-format string=w3663:string)  [unwired: 2 in]
                        n2616 = Concatenate Strings("Set Stroke [mm] :" ("Content"), w3663) -> (w3665:string)
                        n2617 = local read "EVENT LOG"() -> (w3667:string)
                        n2618 = call "Event Log.vi"("Content"=w3665, "EVENT LOG"=w3667) -> ("EVENT LOG"=w3666:string)  [unwired: 8 in, 1 out]
                        n2619 = local write "EVENT LOG"(w3666) -> ()
                      }
                      frame #26 {
                        n2620 = Wait (ms)(milliseconds to wait=u32 50) -> ()  [unwired: 1 out]
                      }
                      frame #27 {
                        n2621 = local read "Set Temp"() -> (w3670:dbl)
                        n2622 = Number To Fractional String(number=w3670, precision (6)=i16 2) -> (F-format string=w3671:string)  [unwired: 2 in]
                        n2623 = Concatenate Strings("Set Temperature [deg C] :" ("Content"), w3671) -> (w3673:string)
                        n2624 = local read "EVENT LOG"() -> (w3675:string)
                        n2625 = call "Event Log.vi"("Content"=w3673, "EVENT LOG"=w3675) -> ("EVENT LOG"=w3674:string)  [unwired: 8 in, 1 out]
                        n2626 = local write "EVENT LOG"(w3674) -> ()
                      }
                      frame #28 {
                        n2627 = Wait (ms)(milliseconds to wait=u32 50) -> ()  [unwired: 1 out]
                      }
                      frame #29 {
                        n2628 = local read "Set Rh"() -> (w3678:dbl)
                        n2629 = Number To Fractional String(number=w3678, precision (6)=i16 2) -> (F-format string=w3679:string)  [unwired: 2 in]
                        n2630 = Concatenate Strings("Set Humidity [%RH] :" ("Content"), w3679) -> (w3681:string)
                        n2631 = local read "EVENT LOG"() -> (w3683:string)
                        n2632 = call "Event Log.vi"("Content"=w3681, "EVENT LOG"=w3683) -> ("EVENT LOG"=w3682:string)  [unwired: 8 in, 1 out]
                        n2633 = local write "EVENT LOG"(w3682) -> ()
                      }
                      frame #30 {
                        n2634 = Wait (ms)(milliseconds to wait=u32 50) -> ()  [unwired: 1 out]
                      }
                      frame #31 {
                        n2635 = local read "test time"() -> (w3686:dbl)
                        n2636 = Number To Fractional String(number=w3686, precision (6)=i16 1) -> (F-format string=w3687:string)  [unwired: 2 in]
                        n2637 = Concatenate Strings("Test Duration [mins] :" ("Content"), w3687) -> (w3689:string)
                        n2638 = local read "EVENT LOG"() -> (w3691:string)
                        n2639 = call "Event Log.vi"("Content"=w3689, "EVENT LOG"=w3691) -> ("EVENT LOG"=w3690:string)  [unwired: 8 in, 1 out]
                        n2640 = local write "EVENT LOG"(w3690) -> ()
                      }
                      frame #32 {
                        w3692 = dbl[] [] ("History Data")
                        w3693 = cluster{"y":dbl, dbl, "y":dbl}[] [] ("History Data")
                        w3694 = FALSE ("Visible")
                        n2641 = property on="Stroke ( mm )" class="WFChart (strict)"("History Data"=w3693) -> ()  [unwired: 2 in, 2 out]
                        n2642 = property on="Temperature ( Deg C )" class="WFChart (strict)"("History Data"=w3692) -> ()  [unwired: 2 in, 2 out]
                        n2643 = property on="Electrical Contact Resistance ( % )" class="WFChart (strict)"("History Data"=w3692) -> ()  [unwired: 2 in, 2 out]
                        n2644 = property on="Coefficient of Friction" class="WFChart (strict)"("History Data"=w3692) -> ()  [unwired: 2 in, 2 out]
                        n2645 = property on="Frictional Force ( N )" class="WFChart (strict)"("History Data"=w3692) -> ()  [unwired: 2 in, 2 out]
                        n2646 = property on="Coefficient of Friction" class="WFChart (strict)"("History Data"=w3692) -> ()  [unwired: 2 in, 2 out]
                        n2647 = property on="Frictional Force ( N )" class="WFChart (strict)"("History Data"=w3692) -> ()  [unwired: 2 in, 2 out]
                        n2648 = property on="Electrical Contact Resistance ( % )" class="WFChart (strict)"("History Data"=w3692) -> ()  [unwired: 2 in, 2 out]
                        n2649 = property on="Stroke ( mm )" class="WFChart (strict)"("History Data"=w3693) -> ()  [unwired: 2 in, 2 out]
                        n2650 = property on="Temperature ( Deg C )" class="WFChart (strict)"("History Data"=w3692) -> ()  [unwired: 2 in, 2 out]
                        n2651 = property on="Service Password Log" class="Str"("Visible"=w3694) -> ()  [unwired: 2 in, 2 out]
                        n2652 = property on="Password 3" class="Clust (strict)"("Visible"=w3694) -> ()  [unwired: 2 in, 2 out]
                      }
                    }
                    "TEST FILE NAM,E SAVED" <- TRUE ("TEST FILE NAM,E SAVED")
                  }
                }
              }
            }
          }
        }
        n2653 = local write "Test \nStatus"(w3081) -> ()
        n2654 = local write "Save"(w3081) -> ()
        n2655 = local read "Main Tab"() -> (w3075:T4)
        n2656 = case shown="True" w3078 {
          frame False {
            n2657 = local read "Rt 3"() -> (w3142:bool)
            n2658 = case shown="True" w3142 {
              frame False {
              }
              frame True {
                n2659 = local write "Rt 3"(FALSE ("Rt 3")) -> ()
              }
            }
            "Rt" <- TRUE ("Rt")
            "Rt 2" <- FALSE ("Rt")
          }
          frame True {
            n2660 = local read "Rt"() -> (w3148:bool)
            n2661 = local write "Rt 2"(TRUE ("Rt 2")) -> ()
            n2662 = case shown="True" w3148 {
              frame False {
              }
              frame True {
                n2663 = local write "Rt"(FALSE ("Rt")) -> ()
              }
            }
            "Rt 3" <- TRUE ("Rt 3")
          }
        }
        n2664 = case shown="\"Acquire\"" w3075 {
          tunnel: w3077 -> [_ w3177]
          frame Default {
            w3176 = 0.0 ("output")
            n2665 = local write "PID-out"(w3176) -> ()
            n2666 = local write "Frequency ( Hz )"(w3176) -> ()
            n2667 = local write "STROKE Initialize"(TRUE ("STROKE Initialize")) -> ()
          }
          frame "Acquire" {
            n2668 = stacked-sequence {
              frame #0 {
                n2669 = local read "Auto Start Test"() -> (w3179:bool)
                n2670 = case shown="True" w3179 {
                  tunnel: "RUN" -> [w3200 w3203]
                  tunnel: [w3200 w3202] -> w3180
                  frame False {
                  }
                  frame True {
                    n2671 = local read "Auto Start Temp"() -> (w3201:bool)
                    n2672 = Or(x=w3203, y=w3201) -> (x .or. y?=w3202:bool)
                  }
                }
                n2673 = local read "clk"() -> (w3199:dbl)
                n2674 = local read "Save"() -> (w3195:bool)
                n2675 = Equal?(x=w3199, y=0.0) -> (x = y?=w3196:bool)
                n2676 = And(x=w3196, y=w3195) -> (x .and. y?=w3197:bool)
                n2677 = Not(x="Engage") -> (.not. x?=w3186:bool)
                n2678 = case shown="False" w3180 {
                  tunnel: [0.0 w3227] -> w3182
                  frame False {
                    (unwired) TRUE ("Visible")
                    n2679 = local read "Auto Start Test"() -> (w3207:bool)
                    n2680 = local write "Start Time"(TRUE ("Start Time")) -> ()
                    n2681 = property on="Stroke 2" class="DigNum (strict)"("Visible"=FALSE) -> ()  [unwired: 2 in, 2 out]
                    n2682 = case shown="False" w3207 {
                      frame False {
                        n2683 = property on="Heater Button" class="Bool (strict)"("DisabledEnum"=T19."Enabled" ("Disabled")) -> ()  [unwired: 2 in, 2 out]
                        n2684 = property on="Humidity" class="Bool (strict)"("DisabledEnum"=T19."Enabled" ("Disabled")) -> ()  [unwired: 2 in, 2 out]
                      }
                      frame True {
                      }
                    }
                    n2685 = case shown="False" "TestCompFlg" {
                      frame False {
                        n2686 = local read "StartFlg"() -> (w3215:bool)
                        n2687 = case shown="True" w3215 {
                          frame False {
                          }
                          frame True {
                            n2688 = stacked-sequence {
                              frame #0 {
                                n2689 = local read "EVENT LOG"() -> (w3219:string)
                                n2690 = call "Event Log.vi"("Content"="Test was interrupted", "EVENT LOG"=w3219) -> ("EVENT LOG"=w3220:string)  [unwired: 8 in, 1 out]
                                n2691 = local write "EVENT LOG"(w3220) -> ()
                                n2692 = property on="RUN" class="Bool (strict)"("Visible"=TRUE) -> ()  [unwired: 2 in, 2 out]
                                n2693 = property on="Auto Start Test" class="Bool (strict)"("Visible"=TRUE) -> ()  [unwired: 2 in, 2 out]
                              }
                              frame #1 {
                                w3223 = FALSE ("StartFlg")
                                n2694 = property on="Heater Button" class="Bool (strict)"("Val(Sgnl)"=FALSE ("Value (Signaling)")) -> ()  [unwired: 2 in, 2 out]
                                n2695 = local write "Heater Button"(w3223) -> ()
                                n2696 = local write "StartFlg"(w3223) -> ()
                                n2697 = local write "Humidity"(w3223) -> ()
                                n2698 = local write "Humidity 2"(TRUE ("Humidity")) -> ()
                              }
                              frame #2 {
                                n2699 = local write "Due Write"("VC;0" ("Command")) -> ()
                              }
                              frame #3 {
                                n2700 = Wait (ms)(milliseconds to wait=u32 1500) -> ()  [unwired: 1 out]
                              }
                              frame #4 {
                                n2701 = local write "Due Write"("HE;0" ("Command")) -> ()
                              }
                            }
                          }
                        }
                      }
                      frame True {
                      }
                    }
                    n2702 = local write "String 14"("Test will autostart once parameters reach the set value." ("String 14")) -> ()
                  }
                  frame True {
                    (unwired) FALSE ("Visible")
                    n2703 = property on="Stroke 2" class="DigNum (strict)"("Visible"=TRUE) -> ()  [unwired: 2 in, 2 out]
                    n2704 = property on="STOP 2" class="Bool (strict)"("Disabled"=u8 2) -> ()  [unwired: 2 in, 2 out]
                    n2705 = local write "String 14"(" Running....." ("String 14")) -> ()
                    n2706 = property on="Heater Button" class="Bool (strict)"("DisabledEnum"=T19."Disabled and Grayed Out" ("Disabled")) -> ()  [unwired: 2 in, 2 out]
                    n2707 = property on="Humidity" class="Bool (strict)"("DisabledEnum"=T19."Disabled and Grayed Out" ("Disabled")) -> ()  [unwired: 2 in, 2 out]
                    n2708 = case shown="True" "Start Time" {
                      selector: "Start Time" -> [_ w3246]
                      frame False {
                      }
                      frame True {
                        n2709 = Not(x=w3246) -> (.not. x?=w3245:bool)
                        n2710 = local write "Start Time"(w3245) -> ()
                        n2711 = local read "EVENT LOG"() -> (w3247:string)
                        n2712 = call "Event Log.vi"("Content"="Test in progress", "EVENT LOG"=w3247) -> ("EVENT LOG"=w3249:string)  [unwired: 8 in, 1 out]
                        n2713 = local write "EVENT LOG"(w3249) -> ()
                      }
                    }
                    n2714 = disable-structure shown="Enabled" {
                      disable-tunnel: [w3238 w3244] -> w3227
                      frame Disabled {
                        n2715 = local read "Set Hz"() -> (w3241:dbl)
                        n2716 = call <vilib>:"Uniform White Noise Waveform.vi"() -> ("signal out"=w3240:waveform(dbl))  [unwired: 10 in, 1 out]
                        n2717 = Random Number (0-1)() -> (number: 0 to 1=w3237:dbl)
                        n2718 = Add(x=w3241, y=w3240) -> (x+y=w3239:waveform(dbl))
                        n2719 = Multiply(x=ext 0.01 ("y"), y=w3237) -> (x*y=w3235:ext)
                        n2720 = Multiply(x=w3239, y=w3235) -> (x*y=w3238:waveform(ext))
                      }
                      frame Enabled {
                        n2721 = call-poly <vilib>:"Random Number (Range).vi"("lower bound (0)"=49.89, "upper bound (100)"=50.8) -> ("number"=w3244:dbl)  [unwired: 9 in]
                      }
                    }
                    "StartFlg" <- TRUE ("StartFlg")
                  }
                }
                n2722 = case shown="True" w3197 {
                  frame False {
                  }
                  frame True {
                    n2723 = local write "clk"(10.0 ("clk")) -> ()
                    n2724 = Get Date/Time In Seconds() -> (seconds since 1Jan1904=w3252:timestamp)
                    n2725 = To Double Precision Float(number=w3252) -> (double precision float=w3250:dbl)
                    n2726 = local write "acq timer"(w3250) -> ()
                    n2727 = local write "act save time"(w3250) -> ()
                  }
                }
                n2728 = call "Elapsed Time"("Time Target (s)"="Countdown", "Reset"=w3186) -> ("Elapsed Time (s)"=w3191:dbl, "Time has Elapsed"=w3189:bool)  [unwired: 10 in, 6 out]
                "Countdown 2" <- w3191
                n2729 = Subtract(x=w3191, y=2.0) -> (x-y=w3194:dbl)
                n2730 = Less?(x=w3194, y="Countdown") -> (x < y?=w3192:bool)
                n2731 = And(x=w3192, y=w3189) -> (x .and. y?=w3188:bool)
                n2732 = case shown="True" w3188 {
                  frame False {
                  }
                  frame True {
                    (unwired) dbl[] [] ("History Data")
                    n2733 = local write "Engage"(FALSE ("Engage")) -> ()
                    n2734 = local write "RUN"(TRUE ("RUN")) -> ()
                    n2735 = local read "Humidity ( %RH )"() -> (→"Rh Before":dbl)
                  }
                }
                n2736 = local read "Test \nStatus"() -> (w3184:bool)
                n2737 = Select(t=w3182, s=w3184, f=0.0) -> (s? t:f=w3183:dbl)
                n2738 = local write "Frequency ( Hz )"(w3183) -> ()
              }
              frame #1 {
                w3275 = 1000000.0 ("x")
                # "HC;1/0\nST;VALUE"
                # "Elapsed time\ncof\nstroke\nAir temp\nTemp\nHumidity"
                # "acq timer\n\nact save time"
                # "convert to microseconds"
                n2739 = local read "COUNT"() -> (w3258:i32)
                n2740 = local read "Rate"() -> (w3271:dbl)
                n2741 = Divide(x=w3275, y=w3271) -> (x/y=w3276:dbl)
                n2742 = Greater Or Equal?(x=w3258, y=250) -> (x >= y?=w3257:bool)
                n2743 = Get Date/Time In Seconds() -> (seconds since 1Jan1904=w3278:timestamp)
                n2744 = case shown="True" w3257 {
                  frame False {
                    n2745 = local read "COUNT"() -> (w3279:i32)
                    n2746 = Increment(x=w3279) -> (x+1=w3280:i32)
                    n2747 = local write "COUNT"(w3280) -> ()
                  }
                  frame True {
                    n2748 = local write "COUNT"(0 ("COUNT")) -> ()
                  }
                }
                n2749 = local read "Samplingtime 2"() -> (w3256:dbl)
                n2750 = local read "act save time"() -> (w3273:dbl)
                n2751 = Divide(x=w3276, y=w3275) -> (x/y=w3274:dbl)
                n2752 = To Double Precision Float(number=w3278) -> (double precision float=w3267:dbl)
                n2753 = Add(x=w3273, y=w3256) -> (x+y=w3272:dbl)
                n2754 = local read "acq timer"() -> (w3277:dbl)
                n2755 = local read "COUNT"() -> (w3260:i32)
                n2756 = Greater Or Equal?(x=w3267, y=w3272) -> (x >= y?=w3255:bool)